vi "UHR-Fleezers Control (host) - 10.3.vi"() -> ()   [LabVIEW 2010] (continued)
  n58 = Divide(x=w183, y=w184) -> (x/y=w182:dbl)
  n59 = Unbundle By Name(w212) -> ("Set 1"=w211:i16, "Set 2"=w210:i16)
  n60 = local read "2D or 1D Scan"() -> (w100:bool)
  n61 = local write "Data points/scans"(w183) -> ()
  n62 = local read "Scan BD"() -> (w201:bool)
  n63 = And(x=w217, y=w218) -> (x .and. y?=w216:cluster{"Set 1":bool, "Set 2":bool})
  n64 = local write "Data points/scan (f/b)"(w186) -> ()
  n65 = Reciprocal(x=w153) -> (1/x=w154:dbl)
  n66 = local read "N Acq Sets (Traps + Fl.)"() -> (w145:i16)
  n67 = local write "N sets should be saved"(w182) -> ()
  n68 = Unbundle By Name(w216) -> ("Set 1"=w220:bool, "Set 2"=w219:bool)
  n69 = local read "Interlace"() -> (w80:bool)
  n70 = Select(t=w87, s=w80, f=w85) -> (s? t:f=w77:u32)
  n71 = local write "Update Count (MCL)"(w77) -> ()
  n72 = local write "Total Counts (ticks)"(w77) -> ()
  n73 = xnode "Invoke Method"("FPGA VI Reference In"=w206, "error in"=w205) -> ("FPGA VI Reference Out"=w98:T19, "error out"=w119:errorcluster)
  n74 = local write "Ave. Period (s)"(w154) -> ()
  n75 = property on="2D or 1D Scan" class="Bool (strict)"("Val(Sgnl)"=w100) -> ()  [unwired: 2 in, 2 out]
  n76 = xnode "Read/Write Control"("FPGA VI Reference In"=w97, "error in"=w119, "ai count"="AI Count (ticks)", "Interlace ON/OFF"=w80, "Number Interlace Cycles"=w79, "AI1 Sets to FIFO"=w221, "FB On/Off Set 1"=w220, "FB On/Off Set 2"=w219, "Interlace Off Parameters"=w78, "FB Setpoint Set 1"=w211, "FB Setpoint Set 2"=w210, "FB Gains Set 1"=w208, "FB Gains Set 2"=w207, "FB output range 1"=w99, "FB output range 2"=w99, "Cycles per step"=w189, "Scan BD"=w201, "Number of scans"=w185, "Scan steps"=w190, "Scan freq.  increment"=w191, "AO1"=w173, "AO2"=w172, "Scan freq.  increment (MCL)"=w166, "Scan steps (MCL)"=w165, "Cycles per step (MCL)"=w164, "Number of scans (MCL)"=w163, "MCL count"=w77, "Cont. Scan (MCL)"=w162, "MCL Scan Axis"=w156, "1D or 2D Scan?"=w100, "N of AI1 Int Acq Sets"=w145, "Freq or Amp switch first"="Freq or Amp switch first", "Freq switch delay"="Freq switch delay", "Amp switch delay"="Amp switch delay", "Swap F1 and F2"="Swap F1 and F2", "APD Acq Rate Count"=w105, "APD to FIFO"=FALSE, "APD Gate Operating Mode"="APD Gate", "APD Gate ON Count"="APD Gate ON Count", "APD Gate OFF Count"="APD Gate OFF Count", "Invert APD Gate"="Invert APD Gate", "DIO count 1 (ticks)"="DIO count 1 (ticks)", "DIO count 2 (ticks)"="DIO count 2 (ticks)", "DIO count 3 (ticks)"="DIO count 3 (ticks)", "APD 1 AO scale factor"="APD 1 AO Mult.", "APD 2 AO scale factor"="APD 2 AO Mult.") -> ("FPGA VI Reference Out"=w72:T19, "error out"=w74:errorcluster)  [unwired: 1 in]
  n77 = local read "Green Laser ON/Interlacing"() -> (w75:bool)
  n78 = local read "Green laser mode"() -> (w76:enum32{"Laser ON", "Laser OFF", "Interlace"})
  n79 = local read "GI Frequency, OFF count"() -> (w68:u32)
  n80 = local read "GI Frequency, ON count"() -> (w67:u32)
  n81 = Multiply(x="Current When FB OFF (%)", y=655.35) -> (x*y=w58:dbl)
  n82 = local read "Green FB Count"() -> (w66:u32)
  n83 = Multiply(x="Green FB Setpoint (mV)", y=3.2767) -> (x*y=w55:dbl)
  n84 = To Unsigned Word Integer(number=w58) -> (unsigned 16bit integer=w56:u16)
  n85 = local read "Invert GI"() -> (w70:bool)
  n86 = To Word Integer(number=w55) -> (16bit integer=w53:i16)
  n87 = case shown="False" w75 {
    tunnel: w76 -> [_ w247]
    tunnel: [enum32{"Laser ON", "Laser OFF", "Interlace"}."Laser OFF" ("Green laser mode") w247] -> w69
    frame False {
    }
    frame True {
    }
  }
  n88 = local read "Trap Pos. AI1 X Pre-scale"() -> (w11:u16)
  n89 = local read "Trap Pos FB Monitor\nT1 or T2"() -> (w18:bool)
  n90 = local read "Trap Pos FB Int Count"() -> (w4:u16)
  n91 = local read "Trap Pos FB Negate Action"() -> (w17:bool)
  n92 = local read "Trap Pos. FB Offset Factor"() -> (w16:i64)
  n93 = local read "Trap Pos. FB Mult Factor"() -> (w15:i64)
  n94 = local read "Trap Pos. FB Gains"() -> (w13:T11)
  n95 = local read "Trap Pos. FB Range"() -> (w14:T12)
  n96 = xnode "Read/Write Control"("FPGA VI Reference In"=w72, "error in"=w74, "Green interlace ON count 2"=w67, "Green interlace OFF count 2"=w68, "Invert GI 2"=w70, "Operating Mode 2"=w69, "Green FB Gains"="Green FB Gains", "Green FB Setpoint"=w53, "Green FB On/Off"="Green FB On/Off", "Current Out"=w56, "Green int current ON count adj"="Green int current ON count adj", "Green FB Count"=w66, "Operating Mode"=w69, "Green interlace OFF count"=w68, "Green interlace ON count"=w67, "Invert GI"=w70, "Trap Pos FB Monitor T1 or T2"=w18, "Trap Pos FB Negate Action"=w17, "Trap Pos. FB Offset Factor"=w16, "Trap Pos. FB Mult Factor"=w15, "Trap Pos. FB Range"=w14, "Trap Pos. FB Gains"=w13, "Force feedback"=FALSE, "AI1 X Scale"=w11, "Trap Pos to FIFO"=TRUE, "Trap Pos FB Int Count"=w4) -> ("FPGA VI Reference Out"=w71:T19, "error out"=w73:errorcluster)
  n97 = xnode "Invoke Method"("FPGA VI Reference In"=w71, "error in"=w73, "Depth"="Trap AI FIFO Depth") -> ("FPGA VI Reference Out"=w21:T19, "error out"=w20:errorcluster)
  n98 = xnode "Invoke Method"("FPGA VI Reference In"=w21, "error in"=w20, "Depth"="Trap Position FIFO Depth") -> ("FPGA VI Reference Out"=w6:T19, "error out"=w5:errorcluster)
  n99 = flat-sequence {
    tunnel: w98 -> [w252]
    tunnel: [w252] -> w97
    tunnel: [w251] -> w96
    tunnel: [w250] -> w95
    tunnel: [w248] -> w93
    tunnel: [w249] -> w94
    frame #0 {
      w249 = T16 {"Minimum"=0.0, "Maximum"=40.0, "Increment"=1.0} ("Min Max Inc")
      w248 = T16 {"Minimum"=0.0, "Maximum"=50.0, "Increment"=1.0} ("Data Entry Limits")
      w251 = T16 {"Minimum"=60.0, "Maximum"=90.0, "Increment"=1.0} ("Min Max Inc")
      w250 = T16 {"Minimum"=0.0, "Maximum"=50.0, "Increment"=1.0} ("Data Entry Limits")
      n100 = property on="BD 2 Frequency 1 (MHz)" class="DigNum (strict)"("Data Range"=w249) -> ()  [unwired: 2 in, 2 out]
      n101 = property on="BD 2 Frequency 3 (MHz)" class="DigNum (strict)"("Data Range"=w249) -> ()  [unwired: 2 in, 2 out]
      n102 = property on="BD 2 Frequency 2 (MHz)" class="DigNum (strict)"("Data Range"=w249) -> ()  [unwired: 2 in, 2 out]
      n103 = property on="BD 1 Frequency 1 (MHz)" class="DigNum (strict)"("Data Range"=w251) -> ()  [unwired: 2 in, 2 out]
      n104 = property on="BD 1 Frequency 2 (MHz)" class="DigNum (strict)"("Data Range"=w251) -> ()  [unwired: 2 in, 2 out]
      n105 = property on="BD 1 Frequency 3 (MHz)" class="DigNum (strict)"("Data Range"=w251) -> ()  [unwired: 2 in, 2 out]
      n106 = property on="BD 2 Amplitude 1 (%)" class="DigNum (strict)"("Data Range"=w248) -> ()  [unwired: 2 in, 2 out]
      n107 = property on="BD 2 Amplitude 2 (%)" class="DigNum (strict)"("Data Range"=w248) -> ()  [unwired: 2 in, 2 out]
      n108 = property on="BD 2 Amplitude 3 (%)" class="DigNum (strict)"("Data Range"=w248) -> ()  [unwired: 2 in, 2 out]
      n109 = property on="BD 1 Amplitude 3 (%)" class="DigNum (strict)"("Data Range"=w250) -> ()  [unwired: 2 in, 2 out]
      n110 = property on="BD 1 Amplitude 2 (%)" class="DigNum (strict)"("Data Range"=w250) -> ()  [unwired: 2 in, 2 out]
      n111 = property on="BD 1 Amplitude 1 (%)" class="DigNum (strict)"("Data Range"=w250) -> ()  [unwired: 2 in, 2 out]
      "X RF Frequency Limits (MHz)" <- w251
      "X RF Amplitude Limits (%)" <- w250
      "Y RF Amplitude Limits (%)" <- w248
      "Y RF Frequency Limits (MHz)" <- w249
    }
  }
  n112 = xnode "Invoke Method"("FPGA VI Reference In"=w6, "error in"=w5) -> ("FPGA VI Reference Out"=w118:T19, "error out"=w117:errorcluster)  [unwired: 1 out]
  n113 = flat-sequence "Initial FPGA Loop Relative Phase Adjustment" {
    tunnel: "Initial Phase Adjustment (AI1)" -> [w263]
    tunnel: "Initial Phase Adjustment (GI)" -> [w262]
    tunnel: w118 -> [w261]
    tunnel: w117 -> [w260]
    tunnel: "Initial Phase Adj. (MCL)" -> [w259]
    tunnel: [w264] -> w127
    tunnel: [w258] -> w123
    tunnel: "Initial Phase Adjustment (APD Acq)" -> [w257]
    tunnel: "Initial Phase Adjustment (APD 1 Gate)" -> [w256]
    tunnel: "Initial Phase Adjustment (Green FB)" -> [w255]
    tunnel: "Initial Phase Adjustment (GI) 2" -> [w254]
    tunnel: "Initial Phase Adjustment (APD 2 Gate)" -> [w253]
    tunnel: w127 -> [w443]
    tunnel: [w444] -> w124
    tunnel: w123 -> [w444]
    tunnel: [w443] -> w122
    tunnel: w124 -> [w447]
    tunnel: w122 -> [w446]
    tunnel: [w449] -> w121
    tunnel: [w448] -> w120
    tunnel: [w636] -> w125
    tunnel: [w637] -> w126
    tunnel: w121 -> [w637]
    tunnel: w120 -> [w636]
    frame #0 {
      n114 = xnode "Read/Write Control"("FPGA VI Reference In"=w261, "error in"=w260, "Phase count adjustment"=w263, "Phase count adjustment (GI)"=w262, "Phase count adjustment (MCL)"=w259, "Phase Count Adjustment (APD Acq)"=w257, "Phase count adjustment (APD 1 Gate)"=w256, "Phase count adjustment (APD 2 Gate)"=w253, "Phase count adjustment (Green FB)"=w255, "Phase count adjustment (GI) 2"=w254) -> ("FPGA VI Reference Out"=w258:T19, "error out"=w264:errorcluster)
    }
    frame #1 {
      n115 = Wait (ms)(milliseconds to wait=u32 100) -> ()  [unwired: 1 out]
    }
    frame #2 {
      w445 = TRUE
      n116 = xnode "Read/Write Control"("FPGA VI Reference In"=w447, "error in"=w446, "+ phase"=w445, "+ phase (GI)"=w445, "+ phase (MCL)"=w445, "+ phase (APD Acq)"=w445, "+ phase (APD 1 Gate)"=w445, "+ phase (APD 2 Gate)"=w445, "+ phase (Green FB)"=w445, "+ phase (GI) 2"=w445) -> ("FPGA VI Reference Out"=w448:T19, "error out"=w449:errorcluster)
    }
    frame #3 {
      n117 = Wait (ms)(milliseconds to wait=u32 100) -> ()  [unwired: 1 out]
    }
  }
  n118 = local read "Phase adj. (Green FB)"() -> (w89:i16)
  n119 = local read "Phase adj. (GI) 2"() -> (w59:i16)
  n120 = local read "Phase adjust (MCL)"() -> (w157:i16)
  n121 = local read "Phase adj. (AI1)"() -> (w159:i16)
  n122 = local read "Phase adj. (GI)"() -> (w158:i16)
  n123 = xnode "Read/Write Control"("FPGA VI Reference In"=w125, "error in"=w126, "Phase count adjustment"=w159, "Phase count adjustment (GI)"=w158, "Phase count adjustment (MCL)"=w157, "Phase Count Adjustment (APD Acq)"="Phase Adj. (APD Acq)", "Phase count adjustment (APD 1 Gate)"="Phase Adj. (APD 1 Gate)", "Phase count adjustment (APD 2 Gate)"="Phase Adj. (APD 2 Gate)", "Phase count adjustment (Green FB)"=w89, "Phase count adjustment (GI) 2"=w59) -> ("FPGA VI Reference Out"=w45:T19, "error out"=w134:errorcluster)
  n124 = call "Initialize RF boards - interlace 3.vi"("error in"=w134, "FPGA VI Reference In"=w45) -> ("error out"=w132:errorcluster, "FPGA VI Reference Out"=w133:T19)
  n125 = call "set RF board frequency - interlace.vi"("Board 2 Frequency Limits"=w94, "Board 1 Frequency Limits"=w96, "error in"=w132, "FPGA VI Reference In"=w133, "Board 2 Frequency 3 (MHz)"="BD 2 Frequency 3 (MHz)", "Board 1 Frequency 3 (MHz)"="BD 1 Frequency 3 (MHz)", "Board 2 Frequency 2 (MHz)"="BD 2 Frequency 2 (MHz)", "Board 2 Frequency 1 (MHz)"="BD 2 Frequency 1 (MHz)", "Board 1 Frequency 2 (MHz)"="BD 1 Frequency 2 (MHz)", "Board 1 Frequency 1  (MHz)"="BD 1 Frequency 1 (MHz)") -> ("error out"=w236:errorcluster, "FPGA VI Reference Out"=w237:T19)
  n126 = call "set RF board amplitude - interlace.vi"("Board 2 Amplitude Limits"=w93, "Board 1 Amplitude Limits"=w95, "error in"=w236, "FPGA VI Reference In"=w237, "Board 2 Amplitude 3 (%)"="BD 2 Amplitude 3 (%)", "Board 1 Amplitude 3 (%)"="BD 1 Amplitude 3 (%)", "Board 2 Amplitude 2 (%)"="BD 2 Amplitude 2 (%)", "Board 2 Amplitude 1 (%)"="BD 2 Amplitude 1 (%)", "Board 1 Amplitude 2 (%)"="BD 1 Amplitude 2 (%)", "Board 1 Amplitude 1 (%)"="BD 1 Amplitude 1 (%)") -> ("error out"=w224:errorcluster, "FPGA VI Reference Out"=w225:T19)
  n127 = flat-sequence {
    tunnel: w225 -> [w646]
    tunnel: w224 -> [w645]
    tunnel: [w644] -> w229
    tunnel: [w643] -> w228
    tunnel: [w688] -> w227
    tunnel: w229 -> [w688]
    tunnel: [w687] -> w226
    tunnel: w228 -> [w687]
    tunnel: w227 -> [w697]
    tunnel: w226 -> [w696]
    tunnel: [w695] -> w8
    tunnel: [w694] -> w7
    frame #0 {
      n128 = local read "Trap 1 (ON/OFF)"() -> (w638:bool)
      n129 = xnode "Read/Write Control"("FPGA VI Reference In"=w646, "error in"=w645, "Direct RF Box  Communication"=FALSE) -> ("FPGA VI Reference Out"=w644:T19, "error out"=w643:errorcluster)
      n130 = local write "Saving..."(FALSE ("Saving Data")) -> ()
      n131 = local write "Stop All"(FALSE ("Stop All")) -> ()
      n132 = local write "Index"(1.0 ("Index")) -> ()
      n133 = property on="Trap 1 ON" class="Bool (strict)"("Value"=w638) -> ()  [unwired: 2 in, 2 out]
      "Manipulating Trap" <- FALSE ("Manipulating Trap")
    }
    frame #1 {
      n134 = local read "Trap 2 (ON/OFF)"() -> (w686:bool)
      n135 = Wait (ms)(milliseconds to wait=u32 10) -> ()  [unwired: 1 out]
      n136 = property on="Trap 2 ON" class="Bool (strict)"("Val(Sgnl)"=w686) -> ()  [unwired: 2 in, 2 out]
    }
    frame #2 {
      n137 = local read "Scan Range (nm)"() -> (w690:dbl)
      n138 = xnode "Read/Write Control"("FPGA VI Reference In"=w697, "error in"=w696, "FPGA Controls  RF Box"=TRUE ("Direct RF Box  Communication")) -> ("FPGA VI Reference Out"=w695:T19, "error out"=w694:errorcluster)
      n139 = call "Update messages.vi"("Message to add"="UHR-Fleezers ready.", "Old message string"="") -> ("New message string"=w693:string)
      n140 = local write "Messages"(w693) -> ()
      n141 = property on="Scan Range (nm)" class="DigNum (strict)"("Val(Sgnl)"=w690) -> ()  [unwired: 2 in, 2 out]
    }
  }
  n142 = Subtract(x="BD 1 Frequency 1 (MHz)", y="BD 1 Frequency 2 (MHz)") -> (x-y=w144:dbl)
  n143 = Subtract(x="BD 2 Frequency 1 (MHz)", y="BD 2 Frequency 2 (MHz)") -> (x-y=w143:dbl)
  n144 = Square(x=w143) -> (x^2=w141:dbl)
  n145 = Square(x=w144) -> (x^2=w142:dbl)
  n146 = Add(x=w142, y=w141) -> (x+y=w140:dbl)
  n147 = Square Root(x=w140) -> (sqrt(x)=w139:dbl)
  n148 = local write "Trap Delta (MHz)"(w139) -> ()
  n149 = call-poly "VISA Configure Serial Port"("VISA resource name"="Sample Chamber Stage Serial Port") -> ("VISA resource name out"=w40:refnum<visa-resource-name>, "error out"=w41:errorcluster)  [unwired: 5 in, 8 out]
  "Stage Control Serial Error" <- w41
  n150 = call "IMAQ Create"("Image Name"="APD 1 Image", "Image Type"=w32) -> ("New Image"=w31:T2)  [unwired: 3 in, 1 out]
  n151 = call "IMAQ Create"("Image Name"="APD 2 Image", "Image Type"=w32) -> ("New Image"=w30:T2)  [unwired: 3 in, 1 out]
  n152 = call "IMAQ Create"("Image Name"="Det. X Image", "Image Type"=w32) -> ("New Image"=w29:T2)  [unwired: 3 in, 1 out]
  n153 = call "IMAQ Create"("Image Name"="Det. Y Image", "Image Type"=w32) -> ("New Image"=w28:T2)  [unwired: 3 in, 1 out]
  n154 = call-poly "VISA Configure Serial Port"("VISA resource name"="Harvard Syringe Pump Serial Port", "baud rate (9600)"=u32 115200, "stop bits (10: 1 bit)"=w25) -> ("VISA resource name out"=w22:refnum<visa-resource-name>, "error out"=w23:errorcluster)  [unwired: 4 in, 7 out]
  n155 = Bundle("New Image"=w31, "New Image"=w30, "New Image"=w29, "New Image"=w28) -> (w27:T22)  [unwired: 1 in]
  n156 = node-c288(i64 1 ("Period"), 1 ("Processor")) -> (w148:T23)  [unwired: 2 out]
  n157 = node-c288(2 ("Processor")) -> (w49:T23)  [unwired: 3 out]
  n158 = node-c288() -> (w37:T23)  [unwired: 4 in]
  n159 = node-c288() -> (w51:T23)  [unwired: 4 out]
  n160 = node-c288(3 ("Processor")) -> (w47:T23)  [unwired: 3 out]
  n161 = disable-structure shown="Disabled" {
    disable-tunnel: [w738 _] -> w204
    disable-tunnel: w8 -> [w737 _]
    frame Disabled {
      n162 = node-c288() -> (w740:T23)  [unwired: 4 out]
      n163 = timed-loop "Rough control of MCL mirror stage (debugging)" {
        tunnel: w737 -> [w743]
        tunnel: [w742] -> w738
        timing: w740 -> [_]
        timing-out: [_] -> w739
        stop <- w742 stop-if-true
        n164 = node-c288() -> ()  [unwired: 2 out]
        n165 = case shown="1" "MCL Mode" {
          tunnel: w743 -> [_ w746 w850]
          frame 0, Default {
          }
          frame 1 {
            n166 = node-c288() -> (w748:T23)  [unwired: 4 out]
            n167 = timed-loop "Oscillate MCL mirror" {
              timing: w748 -> [_]
              timing-out: [_] -> w747
              tunnel: w746 -> [w787]
              i -> [w786]
              stop <- w749 stop-if-true
              n168 = node-c288() -> (w785:i64)  [unwired: 1 out]
              n169 = Multiply(x="AO1", y=32767.0) -> (x*y=w781:dbl)
              n170 = Multiply(x="AO2", y=32767.0) -> (x*y=w776:dbl)
              n171 = Divide(x=w781, y=10.0) -> (x/y=w782:dbl)
              n172 = Divide(x=w776, y=10.0) -> (x/y=w777:dbl)
              n173 = To Word Integer(number=w782) -> (16bit integer=w774:i16)
              n174 = To Word Integer(number=w777) -> (16bit integer=w773:i16)
              n175 = Divide(x=w785, y=i64 1000) -> (x/y=w756:dbl)
              n176 = Multiply(x=w756, y=w786) -> (x*y=w767:dbl)
              n177 = Multiply(x="Osc. freq. (Hz) 2", y=6.283185307179586) -> (x*y=w768:dbl)
              n178 = Multiply(x=w768, y=w767) -> (x*y=w766:dbl)
              n179 = Sine(x=w766) -> (sin(x)=w765:dbl)
              n180 = Multiply(x=w765, y="Osc. amp. (V)") -> (x*y=w763:dbl)
              n181 = Add(x=w763, y="Osc. center (V)") -> (x+y=w761:dbl)
              n182 = Divide(x=w761, y=10.0) -> (x/y=w759:dbl)
              n183 = Multiply(x=w759, y=32767.0) -> (x*y=w754:dbl)
              n184 = Select(t=w754, s="Scan axis", f=w774) -> (s? t:f=w772:dbl)
              n185 = Select(t=w773, s="Scan axis", f=w754) -> (s? t:f=w771:dbl)
              n186 = local read "MCL Mode"() -> (w753:u16)
              n187 = Not Equal?(x=w753, y=u16 1) -> (x != y?=w750:bool)
              n188 = local read "Stop All"() -> (w751:bool)
              n189 = xnode "Read/Write Control"("FPGA VI Reference In"=w787, "AO1"=w772, "AO2"=w771) -> ()  [unwired: 1 in, 2 out]
              n190 = Compound Arithmetic op=OR(w751, w750) -> (w749:bool)
              n191 = node-c288() -> ()  [unwired: 2 out]
            }
            n192 = node-c288(w747) -> ()  [unwired: 1 out]
          }
          frame 2 {
            n193 = case shown="True" "Start Scan" {
              tunnel: w850 -> [_ w862]
              frame False {
              }
              frame True {
                n194 = Subtract(x="End (V)", y="Begin (V)") -> (x-y=w858:dbl)
                n195 = Decrement(x="N Points") -> (x-1=w857:dbl)
                n196 = Divide(x=w858, y=w857) -> (x/y=w855:dbl)
                n197 = for {
                  N: "N Points" -> [_]
                  tunnel: "Begin (V)" -> [w875]
                  tunnel: w862 -> [w867]
                  tunnel: [w866] -> w861 mode=indexing
                  tunnel: w855 -> [w865]
                  tunnel: [w863] -> w854 mode=indexing
                  i -> [w874]
                  n198 = Multiply(x=w865, y=w874) -> (x*y=w873:dbl)
                  n199 = Add(x=w875, y=w873) -> (x+y=w870:dbl)
                  n200 = local read "Scan axis"() -> (w864:bool)
                  n201 = local read "AO1"() -> (w872:dbl)
                  n202 = local read "AO2"() -> (w871:dbl)
                  n203 = Select(t=w870, s=w864, f=w872) -> (s? t:f=w869:dbl)
                  n204 = Select(t=w871, s=w864, f=w870) -> (s? t:f=w868:dbl)
                  n205 = flat-sequence {
                    tunnel: w869 -> [w879]
                    tunnel: w868 -> [w878]
                    tunnel: w867 -> [w876]
                    tunnel: [w946] -> w866
                    tunnel: [w945] -> w863
                    frame #0 {
                      w882 = 10.0 ("y")
                      w877 = 32767.0 ("y")
                      n206 = Multiply(x=w879, y=w877) -> (x*y=w885:dbl)
                      n207 = Multiply(x=w878, y=w877) -> (x*y=w883:dbl)
                      n208 = Divide(x=w885, y=w882) -> (x/y=w886:dbl)
                      n209 = Divide(x=w883, y=w882) -> (x/y=w884:dbl)
                      n210 = To Word Integer(number=w886) -> (16bit integer=w880:i16)
                      n211 = To Word Integer(number=w884) -> (16bit integer=w881:i16)
                      n212 = xnode "Read/Write Control"("FPGA VI Reference In"=w876, "AO1"=w880, "AO2"=w881) -> ()  [unwired: 1 in, 2 out]
                    }
                    frame #1 {
                      n213 = Wait (ms)(milliseconds to wait="DAQ Delay (ms)") -> ()  [unwired: 1 out]
                    }
                    frame #2 {
                      n214 = local read "Slow mean"() -> (w946:dbl)
                      n215 = local read "Sigma"() -> (w945:dbl)
                    }
                  }
                }
                n216 = Bundle("Begin (V)"="Begin (V)", w855, w861) -> (→"MCL Scan":cluster{"Begin (V)":dbl, dbl, dbl[]})  [unwired: 1 out]
                n217 = Bundle("Begin (V)"="Begin (V)", w855, w854) -> (→"MCL Scan 2":cluster{"Begin (V)":dbl, dbl, dbl[]})  [unwired: 1 out]
              }
            }
          }
        }
        n218 = local read "Stop All"() -> (w742:bool)
        n219 = node-c288() -> ()  [unwired: 2 out]
      }
      n220 = node-c288(w739) -> ()  [unwired: 1 out]
    }
    frame Enabled {
    }
  }
  n221 = timed-loop "Acquire Data" {
    tunnel: w8 -> [w1200]
    tunnel: w7 -> [w1199]
    tunnel: [w1230] -> w244
    tunnel: [w1224] -> w242
    timing: w148 -> [_]
    timing-out: [_] -> w147
    tunnel: w27 -> [w1025]
    stop <- "Stop All" stop-if-true
    w1010 = "NI_ChannelName" ("name")
    n222 = node-c288() -> ()  [unwired: 2 out]
    n223 = First Call?() -> (First Call?: T/F=w975:bool)
    n224 = Or(x="Reset", y=w975) -> (x .or. y?=w976:bool)
    n225 = case "Reset data stream" shown="True" w976 {
      tunnel: w1200 -> [w3629 w3637]
      tunnel: w1199 -> [w3628 w3636]
      tunnel: [w3629 w3631] -> w1195
      tunnel: [w3628 w3630] -> w1194
      frame False {
      }
      frame True {
        w3634 = TRUE ("AI to FIFO")
        n226 = local write "Overflow (data lost)"(FALSE ("Overflow (data lost)")) -> ()
        n227 = call "reset FPGA DMA.vi"("error in"=w3636, "FPGA VI Reference In"=w3637) -> ("error out"=w3632:errorcluster, "FPGA VI Reference Out"=w3633:T19)
        n228 = xnode "Read/Write Control"("FPGA VI Reference In"=w3633, "error in"=w3632, "AI to FIFO"=w3634, "APD to FIFO"=w3634) -> ("FPGA VI Reference Out"=w3631:T19, "error out"=w3630:errorcluster)
      }
    }
    n229 = Or(x="Start AOD Scan", y="Trap Raster Scan") -> (x .or. y?=w1145:bool)
    n230 = case "Start AOM raster scan" shown="True" w1145 {
      tunnel: w1195 -> [w2721 w2731]
      tunnel: w1194 -> [w2720 w2730]
      tunnel: [w2721 w2724] -> w1193
      tunnel: [w2720 w2723] -> w1192
      frame False {
      }
      frame True {
        n231 = case shown="True" "Restart DMA? (AOD)" {
          tunnel: [w3142 w3144] -> w2725
          tunnel: [w3141 w3143] -> w2726
          tunnel: w2731 -> [w3142 w3146]
          tunnel: w2730 -> [w3141 w3145]
          frame False {
          }
          frame True {
            n232 = local write "Overflow (data lost)"(FALSE ("Overflow (data lost)")) -> ()
            n233 = call "reset FPGA DMA.vi"("error in"=w3145, "FPGA VI Reference In"=w3146) -> ("error out"=w3143:errorcluster, "FPGA VI Reference Out"=w3144:T19)
          }
        }
        n234 = local write "Trap Raster Scan"(FALSE ("Trap Raster Scan")) -> ()
        n235 = case shown="True" "Move MCL Also?" {
          tunnel: w2726 -> [w2734 w2843]
          tunnel: w2725 -> [w2735 w2844]
          tunnel: [w2733 w2847] -> w2724
          tunnel: [w2732 w2846] -> w2723
          frame False {
            w2736 = TRUE ("AI to FIFO")
            n236 = xnode "Read/Write Control"("FPGA VI Reference In"=w2735, "error in"=w2734, "AI to FIFO"=w2736, "APD to FIFO"=w2736, "Start scan"=w2736) -> ("FPGA VI Reference Out"=w2733:T19, "error out"=w2732:errorcluster)
          }
          frame True {
            w2840 = FALSE ("1D or 2D Scan?")
            w2845 = TRUE ("AI to FIFO")
            # "Count for MCL loop"
            # "N total cycles"
            # "N steps"
            # "V_int"
            n237 = local read "Scan Range (nm)"() -> (w2822:dbl)
            n238 = local read "Number of F/B Scans (AOD)"() -> (w2839:u16)
            n239 = Sign(1:w2822) -> (0:w2821:dbl)
            n240 = Compound Arithmetic op=MULTIPLY(w2822, "MCL Step Position Ratio", "MCL/AOM Scale Tweak") -> (w2826:dbl)
            n241 = Negate(x=w2821) -> (-x=w2818:dbl)
            n242 = Multiply(x=w2818, y="MCL Step Increment (V_int)") -> (x*y=w2820:dbl)
            n243 = Divide(x=w2826, y="MCL X Cal (nm/V)") -> (x/y=w2832:dbl)
            n244 = Multiply(x=32767.0 ("y"), y=w2832) -> (x*y=w2838:dbl)
            n245 = local read "Total Counts (ticks)"() -> (w2823:u32)
            n246 = local read "Cycles/step (AOD)"() -> (w2834:u64)
            n247 = local read "Scan steps (AOD)"() -> (w2835:u64)
            n248 = Divide(x=w2838, y=10.0) -> (x/y=w2831:dbl)
            n249 = Divide(x=w2831, y="MCL Step Increment (V_int)") -> (x/y=w2829:dbl)
            n250 = Absolute Value(x=w2829) -> (abs(x)=w2817:dbl)
            n251 = Compound Arithmetic op=MULTIPLY(w2835, w2834, w2823) -> (w2830:u64)
            n252 = local write "wait to reset values"(w2845) -> ()
            n253 = local write "MCL Scanning"(w2845) -> ()
            n254 = Divide(x=w2830, y=w2817) -> (x/y=w2827:dbl)
            "MCL Count" <- w2827
            n255 = xnode "Read/Write Control"("FPGA VI Reference In"=w2844, "error in"=w2843, "Scan steps (MCL)"=w2817, "Number of scans (MCL)"=w2839, "Cycles per step (MCL)"=u64 1, "Scan freq.  increment (MCL)"=w2820, "1D or 2D Scan?"=w2840, "MCL Scan Axis"=w2840, "Cont. Scan (MCL)"=w2840, "MCL count"=w2827) -> ("FPGA VI Reference Out"=w2842:T19, "error out"=w2841:errorcluster)
            n256 = xnode "Read/Write Control"("FPGA VI Reference In"=w2842, "error in"=w2841, "AI to FIFO"=w2845, "APD to FIFO"=w2845, "Start scan"=w2845, "Start scan (MCL)"=w2845) -> ("FPGA VI Reference Out"=w2847:T19, "error out"=w2846:errorcluster)
          }
        }
        "Raster Scanning..." <- TRUE ("Scanning...")
      }
    }
    n257 = And(x="Save scans", y=w1145) -> (x .and. y?=w1191:bool)
    n258 = Compound Arithmetic op=OR("Start MCL Scan", "Confocal Image", "Confocal Linescan") -> (w1143:bool)
    n259 = And(x="Save Data (MCL)", y=w1143) -> (x .and. y?=w1190:bool)
    n260 = case "Start MCL raster scan" shown="True" w1143 {
      tunnel: w1193 -> [w2062 w2077]
      tunnel: w1192 -> [w2061 w2076]
      tunnel: [w2062 w2072] -> w1023
      tunnel: [w2061 w2071] -> w1022
      tunnel: [FALSE w2070] -> w1176
      tunnel: "Start MCL Scan" -> [_ w2065]
      tunnel: "Confocal Image" -> [_ w2064]
      tunnel: "Confocal Linescan" -> [_ _]
      frame False {
      }
      frame True {
        w2070 = TRUE
        n261 = case shown="True" "Restart DMA? (MCL)" {
          tunnel: [w2322 w2324] -> w2075
          tunnel: [w2321 w2323] -> w2074
          tunnel: w2077 -> [w2322 w2327]
          tunnel: w2076 -> [w2321 w2326]
          frame False {
          }
          frame True {
            n262 = call "reset FPGA DMA.vi"("error in"=w2326, "FPGA VI Reference In"=w2327) -> ("error out"=w2323:errorcluster, "FPGA VI Reference Out"=w2324:T19)